vi "Dresden R2R Sputter 03.02.2018 IY24.vi"() -> ()   [LabVIEW 2009] (continued)
                    frame #0 {
                    }
                    frame #1 {
                      # "Hata mesajı"
                      n13036 = local write "Semi"(TRUE ("Semi")) -> ()
                    }
                  }
                  n13037 = local read "Routine_check_transfer"() -> (w19690:bool)
                  n13038 = local read "Semi"() -> (w19692:bool)
                  n13039 = Not(x=w19690) -> (.not. x?=w19691:bool)
                  n13040 = Or(x=w19691, y=w19692) -> (x .or. y?=w19693:bool)
                }
              }
              frame #2 {
                n13041 = Wait (ms)(milliseconds to wait=u32 500) -> ()  [unwired: 1 out]
              }
            }
          }
          frame #2 {
            # "STARTED UP CH3"
            n13042 = disable-structure shown="Disabled" {
              frame #0 {
                n13043 = local read "Semi"() -> (w19700:bool)
                n13044 = case shown="False" w19700 {
                  frame #0 {
                    n13045 = local read "started_up_ch3"() -> (w19701:bool)
                    n13046 = case shown="False" w19701 {
                      frame #0 {
                        n13047 = stacked-sequence {
                          frame #0 {
                            n13048 = local read "Semi"() -> (w19702:bool)
                            n13049 = case shown="False" w19702 {
                              frame #0 {
                                n13050 = local write "Start_up_ch3"(TRUE ("Start_up_ch2")) -> ()
                              }
                              frame #1 {
                              }
                            }
                          }
                          frame #1 {
                            n13051 = local read "Semi"() -> (w19704:bool)
                            n13052 = case shown="False" w19704 {
                              frame #0 {
                                n13053 = Wait (ms)(milliseconds to wait=u32 16000) -> ()  [unwired: 1 out]
                              }
                              frame #1 {
                              }
                            }
                          }
                          frame #2 {
                            n13054 = local read "Semi"() -> (w19706:bool)
                            n13055 = case shown="False" w19706 {
                              frame #0 {
                                n13056 = while {
                                i -> [w19711]
                                stop <- w19708 stop-if-true
                                n13057 = Greater?(x=w19711, y=80) -> (0:w19709:bool)
                                n13058 = local read "started_up_ch3"() -> (w19707:bool)
                                n13059 = case shown="True" w19709 {
                                frame #0 {
                                }
                                frame #1 {
                                n13060 = local write "Semi"(TRUE ("Semi")) -> ()
                                n13061 = local write "Error Message"("Chamber 1 Pressure is not suitable  \nfor transfer process!\nPlease check connections." ("Error Message")) -> ()
                                }
                                }
                                n13062 = case shown="False" w19707 {
                                tunnel: [FALSE TRUE] -> w19708
                                frame #0 {
                                n13063 = Wait Until Next ms Multiple(millisecond multiple=u32 200) -> ()  [unwired: 1 out]
                                }
                                frame #1 {
                                }
                                }
                                }
                              }
                              frame #1 {
                              }
                            }
                          }
                          frame #3 {
                            n13064 = local read "Semi"() -> (w19717:bool)
                            n13065 = case shown="False" w19717 {
                              frame #0 {
                                n13066 = local write "CH1_2_trns_0"(TRUE ("CH1_2_trns_0")) -> ()
                                n13067 = Wait (ms)(milliseconds to wait=u32 1000) -> ()  [unwired: 1 out]
                              }
                              frame #1 {
                              }
                            }
                          }
                        }
                      }
                      frame #1 {
                      }
                    }
                  }
                  frame #1 {
                  }
                }
              }
              frame #1 {
              }
            }
          }
          frame #3 {
            # "STARTED UP CH2"
            n13068 = disable-structure shown="Disabled" {
              frame #0 {
                n13069 = local read "Semi"() -> (w19720:bool)
                n13070 = case shown="False" w19720 {
                  frame #0 {
                    n13071 = local read "started_up_ch2"() -> (w19721:bool)
                    n13072 = case shown="False" w19721 {
                      frame #0 {
                        n13073 = stacked-sequence {
                          frame #0 {
                            n13074 = local read "Semi"() -> (w19722:bool)
                            n13075 = case shown="False" w19722 {
                              frame #0 {
                                n13076 = local write "Start_up_ch2"(TRUE ("Start_up_ch2")) -> ()
                              }
                              frame #1 {
                              }
                            }
                          }
                          frame #1 {
                            n13077 = local read "Semi"() -> (w19724:bool)
                            n13078 = case shown="False" w19724 {
                              frame #0 {
                                n13079 = Wait (ms)(milliseconds to wait=u32 18000) -> ()  [unwired: 1 out]
                              }
                              frame #1 {
                              }
                            }
                          }
                          frame #2 {
                            n13080 = local read "Semi"() -> (w19726:bool)
                            n13081 = case shown="False" w19726 {
                              frame #0 {
                                n13082 = while {
                                i -> [w19731]
                                stop <- w19728 stop-if-true
                                n13083 = Greater?(x=w19731, y=90) -> (0:w19729:bool)
                                n13084 = local read "started_up_ch2"() -> (w19727:bool)
                                n13085 = case shown="True" w19729 {
                                frame #0 {
                                }
                                frame #1 {
                                n13086 = local write "Semi"(TRUE ("Semi")) -> ()
                                n13087 = local write "Error Message"("Chamber 2 Pressure is not suitable  \nfor transfer process!\nPlease check connections." ("Error Message")) -> ()
                                }
                                }
                                n13088 = case shown="False" w19727 {
                                tunnel: [FALSE TRUE] -> w19728
                                frame #0 {
                                n13089 = Wait Until Next ms Multiple(millisecond multiple=u32 200) -> ()  [unwired: 1 out]
                                }
                                frame #1 {
                                }
                                }
                                }
                              }
                              frame #1 {
                              }
                            }
                          }
                          frame #3 {
                            n13090 = local read "Semi"() -> (w19737:bool)
                            n13091 = case shown="False" w19737 {
                              frame #0 {
                                n13092 = local write "CH1_2_trns_1"(TRUE ("CH1_2_trns_0")) -> ()
                                n13093 = Wait (ms)(milliseconds to wait=u32 1000) -> ()  [unwired: 1 out]
                              }
                              frame #1 {
                              }
                            }
                          }
                        }
                      }
                      frame #1 {
                      }
                    }
                  }
                  frame #1 {
                  }
                }
              }
              frame #1 {
              }
            }
          }
          frame #4 {
            # "TRNS GV-BP OPEN"
            n13094 = local read "Semi"() -> (w19740:bool)
            n13095 = case shown="False" w19740 {
              frame #0 {
                n13096 = stacked-sequence {
                  frame #0 {
                    n13097 = local read "Semi"() -> (w19741:bool)
                    n13098 = case shown="False" w19741 {
                      frame #0 {
                        n13099 = while {
                          i -> [w19748]
                          stop <- w19743 stop-if-true
                          n13100 = Greater?(x=w19748, y=50) -> (0:w19746:bool)
                          n13101 = local read "Ch2_trns_gv_bp2_di"() -> (w19742:bool)
                          n13102 = case shown="True" w19746 {
                            frame #0 {
                            }
                            frame #1 {
                              n13103 = local write "Semi"(TRUE ("Semi")) -> ()
                              n13104 = local write "Error Message"("Transfer process was cancelled.\nPlease check CH1-Trns-GV connections." ("Error Message")) -> ()
                            }
                          }
                          n13105 = case shown="False" w19742 {
                            tunnel: [FALSE TRUE] -> w19745
                            frame #0 {
                              n13106 = Wait Until Next ms Multiple(millisecond multiple=u32 200) -> ()  [unwired: 1 out]
                              n13107 = local write "Ch2_trns_gv_bp2_do"(TRUE ("Ch1_pet_cool_up_do")) -> ()
                            }
                            frame #1 {
                            }
                          }
                          n13108 = local read "Semi"() -> (w19744:bool)
                          n13109 = Or(x=w19745, y=w19744) -> (x .or. y?=w19743:bool)
                        }
                      }
                      frame #1 {
                      }
                    }
                  }
                  frame #1 {
                    n13110 = local read "Semi"() -> (w19755:bool)
                    n13111 = case shown="False" w19755 {
                      frame #0 {
                        n13112 = Wait (ms)(milliseconds to wait=u32 500) -> ()  [unwired: 1 out]
                      }
                      frame #1 {
                      }
                    }
                  }
                  frame #2 {
                    n13113 = local read "Semi"() -> (w19757:bool)
                    n13114 = case shown="False" w19757 {
                      frame #0 {
                        n13115 = while {
                          i -> [w19764]
                          stop <- w19759 stop-if-true
                          n13116 = Greater?(x=w19764, y=50) -> (0:w19762:bool)
                          n13117 = local read "Ch3_Trns_gv_bp_di"() -> (w19758:bool)
                          n13118 = case shown="True" w19762 {
                            frame #0 {
                            }
                            frame #1 {
                              n13119 = local write "Semi"(TRUE ("Semi")) -> ()
                              n13120 = local write "Error Message"("Transfer process was cancelled.\nPlease check CH1-Trns-GV connections." ("Error Message")) -> ()
                            }
                          }
                          n13121 = case shown="False" w19758 {
                            tunnel: [FALSE TRUE] -> w19761
                            frame #0 {
                              n13122 = local write "Ch3_Trns_gv_bp_do"(TRUE ("Ch1_pet_cool_up_do")) -> ()
                              n13123 = Wait Until Next ms Multiple(millisecond multiple=u32 200) -> ()  [unwired: 1 out]
                            }
                            frame #1 {
                            }
                          }
                          n13124 = local read "Semi"() -> (w19760:bool)
                          n13125 = Or(x=w19761, y=w19760) -> (x .or. y?=w19759:bool)
                        }
                      }
                      frame #1 {
                      }
                    }
                  }
                  frame #3 {
                    n13126 = local read "Semi"() -> (w19771:bool)
                    n13127 = case shown="False" w19771 {
                      frame #0 {
                        n13128 = Wait (ms)(milliseconds to wait=u32 500) -> ()  [unwired: 1 out]
                      }
                      frame #1 {
                      }
                    }
                  }
                }
              }
              frame #1 {
              }
            }
          }
          frame #5 {
            # "TRNS GV OPEN"
            n13129 = local read "Semi"() -> (w19773:bool)
            n13130 = case shown="False" w19773 {
              frame #0 {
                n13131 = stacked-sequence {
                  frame #0 {
                    n13132 = local read "Semi"() -> (w19774:bool)
                    n13133 = case shown="False" w19774 {
                      frame #0 {
                        n13134 = local write "Ch2_Trns_gv_close_do"(FALSE ("Ch1_pet_cool_up_do")) -> ()
                      }
                      frame #1 {
                      }
                    }
                  }
                  frame #1 {
                    n13135 = local read "Semi"() -> (w19776:bool)
                    n13136 = case shown="False" w19776 {
                      frame #0 {
                        n13137 = while {
                          i -> [w19783]
                          stop <- w19778 stop-if-true
                          n13138 = Greater?(x=w19783, y=500) -> (0:w19781:bool)
                          n13139 = local read "Ch2_Trns_gv_open_di"() -> (w19777:bool)
                          n13140 = case shown="True" w19781 {
                            frame #0 {
                            }
                            frame #1 {
                              n13141 = local write "Semi"(TRUE ("Semi")) -> ()
                              n13142 = local write "Error Message"("Transfer process was cancelled.\nPlease check CH1-Trns-GV connections." ("Error Message")) -> ()
                            }
                          }
                          n13143 = case shown="False" w19777 {
                            tunnel: [FALSE TRUE] -> w19780
                            frame #0 {
                              n13144 = Wait Until Next ms Multiple(millisecond multiple=u32 200) -> ()  [unwired: 1 out]
                              n13145 = local write "Ch2_Trns_gv_open_do"(TRUE ("Ch1_pet_cool_up_do")) -> ()
                            }
                            frame #1 {
                            }
                          }
                          n13146 = local read "Semi"() -> (w19779:bool)
                          n13147 = Or(x=w19780, y=w19779) -> (x .or. y?=w19778:bool)
                        }
                      }
                      frame #1 {
                      }
                    }
                  }
                  frame #2 {
                    n13148 = local read "Semi"() -> (w19790:bool)
                    n13149 = case shown="False" w19790 {
                      frame #0 {
                        n13150 = local write "CH1_2trns_2"(TRUE ("CH1_2trns_5")) -> ()
                        n13151 = Wait (ms)(milliseconds to wait=u32 500) -> ()  [unwired: 1 out]
                      }
                      frame #1 {
                      }
                    }
                  }
                }
              }
              frame #1 {
              }
            }
          }
          frame #6 {
            # "TRNS GV control Trnsgv 2_3"
            n13152 = local read "Semi"() -> (w19793:bool)
            n13153 = case shown="False" w19793 {
              frame #0 {
                n13154 = stacked-sequence {
                  frame #0 {
                    n13155 = local read "Semi"() -> (w19794:bool)
                    n13156 = case shown="False" w19794 {
                      frame #0 {
                        n13157 = while {
                          i -> [w19801]
                          stop <- w19796 stop-if-true
                          n13158 = Greater?(x=w19801, y=50) -> (0:w19799:bool)
                          n13159 = local read "Ch2_TGV_control_di"() -> (w19795:bool)
                          n13160 = case shown="True" w19799 {
                            frame #0 {
                            }
                            frame #1 {
                              n13161 = local write "Semi"(TRUE ("Semi")) -> ()
                              n13162 = local write "Error Message"("Transfer process was cancelled.\nPlease check TRNS-GV connections." ("Error Message")) -> ()
                            }
                          }
                          n13163 = case shown="True" w19795 {
                            tunnel: [TRUE FALSE] -> w19798
                            frame #0 {
                            }
                            frame #1 {
                              n13164 = Wait Until Next ms Multiple(millisecond multiple=u32 200) -> ()  [unwired: 1 out]
                              n13165 = local write "Ch2_TGV_control_do"(FALSE ("Ch1_pet_cool_up_do")) -> ()
                            }
                          }
                          n13166 = local read "Semi"() -> (w19797:bool)
                          n13167 = Or(x=w19798, y=w19797) -> (x .or. y?=w19796:bool)
                        }
                      }
                      frame #1 {
                      }
                    }
                  }
                  frame #1 {
                    n13168 = local read "Semi"() -> (w19808:bool)
                    n13169 = case shown="False" w19808 {
                      frame #0 {
                        n13170 = local write "CH1_2trns_3"(TRUE ("CH1_2trns_5")) -> ()
                        n13171 = Wait (ms)(milliseconds to wait=u32 500) -> ()  [unwired: 1 out]
                      }
                      frame #1 {
                      }
                    }
                  }
                }
              }
              frame #1 {
              }
            }
          }
          frame #7 {
            # "TRNS GV control Trnsgv 2_3"
            n13172 = local read "Semi"() -> (w19811:bool)
            n13173 = case shown="False" w19811 {
              frame #0 {
                n13174 = stacked-sequence {
                  frame #0 {
                    n13175 = local read "Semi"() -> (w19812:bool)
                    n13176 = case shown="False" w19812 {
                      frame #0 {
                        n13177 = while {
                          i -> [w19819]
                          stop <- w19814 stop-if-true
                          n13178 = Greater?(x=w19819, y=50) -> (0:w19817:bool)
                          n13179 = local read "Ch1_Trns_interlock_di"() -> (w19813:bool)
                          n13180 = case shown="True" w19817 {
                            frame #0 {
                            }
                            frame #1 {
                              n13181 = local write "Semi"(TRUE ("Semi")) -> ()
                              n13182 = local write "Error Message"("Transfer process was cancelled.\nPlease check TRNS-GV connections." ("Error Message")) -> ()
                            }
                          }
                          n13183 = case shown="False" w19813 {
                            tunnel: [w19821 TRUE] -> w19816
                            frame #0 {
                              n13184 = local read "Ch1_TGV_control_di"() -> (w19820:bool)
                              n13185 = case shown="False" w19820 {
                                tunnel: [FALSE TRUE] -> w19821
                                frame #0 {
                                n13186 = Wait Until Next ms Multiple(millisecond multiple=u32 200) -> ()  [unwired: 1 out]
                                n13187 = local write "Ch1_TGV_control_do"(TRUE ("Ch1_pet_cool_up_do")) -> ()
                                }
                                frame #1 {
                                }
                              }
                            }
                            frame #1 {
                            }
                          }
                          n13188 = local read "Semi"() -> (w19815:bool)
                          n13189 = Or(x=w19816, y=w19815) -> (x .or. y?=w19814:bool)
                        }
                      }
                      frame #1 {
                      }
                    }
                  }
                  frame #1 {
                    n13190 = local read "Semi"() -> (w19829:bool)
                    n13191 = case shown="False" w19829 {
                      frame #0 {
                        n13192 = local write "CH1_2trns_3"(TRUE ("CH1_2trns_5")) -> ()
                        n13193 = Wait (ms)(milliseconds to wait=u32 500) -> ()  [unwired: 1 out]
                      }
                      frame #1 {
                      }
                    }
                  }
                }
              }
              frame #1 {
              }
            }
          }
          frame #8 {
            # "TRNS GV control Trnsgv 3_4"
            n13194 = local read "Semi"() -> (w19832:bool)
            n13195 = case shown="False" w19832 {
              frame #0 {
                n13196 = stacked-sequence {
                  frame #0 {
                    n13197 = local read "Semi"() -> (w19833:bool)
                    n13198 = case shown="False" w19833 {
                      frame #0 {
                        n13199 = while {
                          i -> [w19840]
                          stop <- w19835 stop-if-true
                          n13200 = Greater?(x=w19840, y=50) -> (0:w19838:bool)
                          n13201 = local read "Ch3_Trns_interlock_di"() -> (w19834:bool)
                          n13202 = case shown="True" w19838 {
                            frame #0 {
                            }
                            frame #1 {
                              n13203 = local write "Semi"(TRUE ("Semi")) -> ()
                              n13204 = local write "Error Message"("Transfer process was cancelled.\nPlease check TRNS-GV connections." ("Error Message")) -> ()
                            }
                          }
                          n13205 = case shown="False" w19834 {
                            tunnel: [w19842 TRUE] -> w19837
                            frame #0 {
                              n13206 = local read "Ch3_TGV_control_di"() -> (w19841:bool)
                              n13207 = case shown="False" w19841 {
                                tunnel: [FALSE TRUE] -> w19842
                                frame #0 {
                                n13208 = Wait Until Next ms Multiple(millisecond multiple=u32 200) -> ()  [unwired: 1 out]
                                n13209 = local write "Ch3_TGV_control_do"(TRUE ("Ch1_pet_cool_up_do")) -> ()
                                }
                                frame #1 {
                                }
                              }
                            }
                            frame #1 {
                            }
                          }
                          n13210 = local read "Semi"() -> (w19836:bool)
                          n13211 = Or(x=w19837, y=w19836) -> (x .or. y?=w19835:bool)
                        }
                      }
                      frame #1 {
                      }
                    }
                  }
                  frame #1 {
                    n13212 = local read "Semi"() -> (w19850:bool)
                    n13213 = case shown="False" w19850 {
                      frame #0 {
                        n13214 = local write "CH1_2trns_4"(TRUE ("CH1_2trns_5")) -> ()
                        n13215 = Wait (ms)(milliseconds to wait=u32 500) -> ()  [unwired: 1 out]
                      }
                      frame #1 {
                      }
                    }
                  }
                }
              }
              frame #1 {
              }
            }
          }
          frame #9 {
            # "Right slow deactive"
            n13216 = local read "Semi"() -> (w19853:bool)
            n13217 = case shown="False" w19853 {
              frame #0 {
                n13218 = stacked-sequence {
                  frame #0 {
                    n13219 = local read "Semi"() -> (w19854:bool)
                    n13220 = case shown="False" w19854 {
                      frame #0 {
                        n13221 = while {
                          i -> [w19857]
                          stop <- w19858 stop-if-true
                          n13222 = Greater?(x=w19857, y=50) -> (0:w19855:bool)
                          n13223 = local read "Cnt_Right_slow_di"() -> (w19861:bool)
                          n13224 = case shown="True" w19855 {
                            frame #0 {
                            }
                            frame #1 {
                              n13225 = local write "Semi"(TRUE ("Semi")) -> ()
                              n13226 = local write "Error Message"("Transfer process was\ncancelled.Please check right slow sensor." ("Error Message")) -> ()
                            }
                          }
                          n13227 = case shown="False" w19861 {
                            tunnel: [FALSE ("Ch1_pet_cool_up_do") TRUE ("Ch1_pet_cool_up_do")] -> w19860
                            frame #0 {
                              n13228 = Wait Until Next ms Multiple(millisecond multiple=u32 200) -> ()  [unwired: 1 out]
                              n13229 = local write "Cnt_Right_slow_do"(TRUE ("Ch1_pet_cool_up_do")) -> ()
                            }
                            frame #1 {
                            }
                          }
                          n13230 = local read "Semi"() -> (w19859:bool)
                          n13231 = Or(x=w19860, y=w19859) -> (x .or. y?=w19858:bool)
                        }
                      }
                      frame #1 {
                      }
                    }
                  }
                  frame #1 {
                    n13232 = local read "Semi"() -> (w19868:bool)
                    n13233 = case shown="False" w19868 {
                      frame #0 {
                        n13234 = local write "CH1_2trns_5"(TRUE ("CH1_2trns_7")) -> ()
                        n13235 = Wait (ms)(milliseconds to wait=u32 500) -> ()  [unwired: 1 out]
                      }
                      frame #1 {
                      }
                    }
                  }
                }
              }
              frame #1 {
              }
            }
          }
          frame #10 {
            # "Right limit deactive"
            n13236 = local read "Semi"() -> (w19871:bool)
            n13237 = case shown="False" w19871 {
              frame #0 {
                n13238 = stacked-sequence {
                  frame #0 {
                    n13239 = local read "Semi"() -> (w19872:bool)
                    n13240 = case shown="False" w19872 {
                      frame #0 {
                        n13241 = while {
                          i -> [w19873]
                          stop <- w19877 stop-if-true
                          n13242 = Greater?(x=w19873, y=50) -> (0:w19875:bool)
                          n13243 = local read "Cnt_Right_limit_di"() -> (w19879:bool)
                          n13244 = case shown="True" w19875 {
                            frame #0 {
                            }
                            frame #1 {
                              n13245 = local write "Semi"(TRUE ("Semi")) -> ()
                              n13246 = local write "Error Message"("Transfer process was\ncancelled.Please check right limit sensor." ("Error Message")) -> ()
                            }
                          }
                          n13247 = case shown="False" w19879 {
                            tunnel: [FALSE ("Ch1_pet_cool_up_do") TRUE ("Ch1_pet_cool_up_do")] -> w19878
                            frame #0 {
                              n13248 = Wait Until Next ms Multiple(millisecond multiple=u32 200) -> ()  [unwired: 1 out]
                              n13249 = local write "Cnt_Right_limit_do"(TRUE ("Ch1_pet_cool_up_do")) -> ()
                            }
                            frame #1 {
                            }
                          }
                          n13250 = local read "Semi"() -> (w19876:bool)
                          n13251 = Or(x=w19878, y=w19876) -> (x .or. y?=w19877:bool)
                        }
                      }
                      frame #1 {
                      }
                    }
                  }
                  frame #1 {
                    n13252 = local read "Semi"() -> (w19886:bool)
                    n13253 = case shown="False" w19886 {
                      frame #0 {
                        n13254 = local write "CH1_2trns_6"(TRUE ("CH1_2trns_7")) -> ()
                        n13255 = Wait (ms)(milliseconds to wait=u32 500) -> ()  [unwired: 1 out]
                      }
                      frame #1 {
                      }
                    }
                  }
                }
              }
              frame #1 {
              }
            }
          }
          frame #11 {
            # "Left slow deactive"
            n13256 = local read "Semi"() -> (w19889:bool)
            n13257 = case shown="False" w19889 {
              frame #0 {
                n13258 = stacked-sequence {
                  frame #0 {
                    n13259 = local read "Semi"() -> (w19890:bool)
                    n13260 = case shown="False" w19890 {
                      frame #0 {
                        n13261 = while {
                          i -> [w19891]
                          stop <- w19895 stop-if-true
                          n13262 = Greater?(x=w19891, y=50) -> (0:w19893:bool)
                          n13263 = local read "Cnt_Left_slow_di"() -> (w19897:bool)
                          n13264 = case shown="True" w19893 {
                            frame #0 {
                            }
                            frame #1 {
                              n13265 = local write "Semi"(TRUE ("Semi")) -> ()
                              n13266 = local write "Error Message"("Transfer process was\ncancelled.Please check left slow sensor." ("Error Message")) -> ()
                            }
                          }
                          n13267 = case shown="False" w19897 {
                            tunnel: [FALSE ("Ch1_pet_cool_up_do") TRUE ("Ch1_pet_cool_up_do")] -> w19896
                            frame #0 {
                              n13268 = Wait Until Next ms Multiple(millisecond multiple=u32 200) -> ()  [unwired: 1 out]
                              n13269 = local write "Cnt_Left_slow_do"(TRUE ("Ch1_pet_cool_up_do")) -> ()
                            }
                            frame #1 {
                            }
                          }
                          n13270 = local read "Semi"() -> (w19894:bool)
                          n13271 = Or(x=w19896, y=w19894) -> (x .or. y?=w19895:bool)
                        }
                      }
                      frame #1 {
                      }
                    }
                  }
                  frame #1 {
                    n13272 = local read "Semi"() -> (w19904:bool)
                    n13273 = case shown="False" w19904 {
                      frame #0 {
                        n13274 = local write "CH1_2trns_7"(TRUE ("CH1_2trns_6b")) -> ()
                        n13275 = Wait (ms)(milliseconds to wait=u32 500) -> ()  [unwired: 1 out]
                      }
                      frame #1 {
                      }
                    }
                  }
                }
              }
              frame #1 {
              }
            }
          }
          frame #12 {
            # "Left limit deactive"
            n13276 = local read "Semi"() -> (w19907:bool)
            n13277 = case shown="False" w19907 {
              frame #0 {
                n13278 = stacked-sequence {
                  frame #0 {
                    n13279 = local read "Semi"() -> (w19908:bool)
                    n13280 = case shown="False" w19908 {
                      frame #0 {
                        n13281 = while {
                          i -> [w19909]
                          stop <- w19913 stop-if-true
                          n13282 = Greater?(x=w19909, y=50) -> (0:w19911:bool)
                          n13283 = local read "Cnt_Left_limit_di"() -> (w19915:bool)
                          n13284 = case shown="True" w19911 {
                            frame #0 {
                            }
                            frame #1 {
                              n13285 = local write "Semi"(TRUE ("Semi")) -> ()
                              n13286 = local write "Error Message"("Transfer process was\ncancelled.Please check left limit sensor." ("Error Message")) -> ()
                            }
                          }
                          n13287 = case shown="False" w19915 {
                            tunnel: [FALSE ("Ch1_pet_cool_up_do") TRUE ("Ch1_pet_cool_up_do")] -> w19914
                            frame #0 {
                              n13288 = Wait Until Next ms Multiple(millisecond multiple=u32 200) -> ()  [unwired: 1 out]
                              n13289 = local write "Cnt_Left_limit_do"(TRUE ("Ch1_pet_cool_up_do")) -> ()
                            }
                            frame #1 {
                            }
                          }
                          n13290 = local read "Semi"() -> (w19912:bool)
                          n13291 = Or(x=w19914, y=w19912) -> (x .or. y?=w19913:bool)
                        }
                      }
                      frame #1 {
                      }
                    }
                  }
                  frame #1 {
                    n13292 = local read "Semi"() -> (w19922:bool)
                    n13293 = case shown="False" w19922 {
                      frame #0 {
                        n13294 = local write "CH1_2trns_8"(TRUE ("CH1_2trns_6c")) -> ()
                        n13295 = Wait (ms)(milliseconds to wait=u32 500) -> ()  [unwired: 1 out]
                      }
                      frame #1 {
                      }
                    }
                  }
                }
              }
              frame #1 {
              }
            }
          }
          frame #13 {
            # "Casette Direction"
            n13296 = local read "Semi"() -> (w19925:bool)
            n13297 = case shown="False" w19925 {
              frame #0 {
                n13298 = stacked-sequence {
                  frame #0 {
                    n13299 = local read "Semi"() -> (w19926:bool)
                    n13300 = case shown="False" w19926 {
                      frame #0 {
                        n13301 = while {
                          i -> [w19932]
                          stop <- w19927 stop-if-true
                          n13302 = Greater?(x=w19932, y=50) -> (0:w19933:bool)
                          n13303 = case shown="True" w19933 {
                            frame #0 {
                            }
                            frame #1 {
                              n13304 = local write "Semi"(TRUE ("Semi")) -> ()
                              n13305 = local write "Error Message"("Transfer process was cancelled.\nPlease check Casette Direction connections." ("Error Message")) -> ()
                            }
                          }
                          n13306 = local read "Casette_servo_left_direction_di"() -> (w19930:bool)
                          n13307 = case shown="True" w19930 {
                            tunnel: [TRUE ("Casette_servo_left_direction_do") FALSE ("Casette_servo_left_direction_do")] -> w19929
                            frame #0 {
                            }
                            frame #1 {
                              n13308 = Wait Until Next ms Multiple(millisecond multiple=u32 200) -> ()  [unwired: 1 out]
                              n13309 = local write "Casette_servo_left_direction_do"(FALSE ("Casette_servo_left_direction_do")) -> ()
                            }
                          }
                          n13310 = local read "Semi"() -> (w19928:bool)
                          n13311 = Or(x=w19929, y=w19928) -> (x .or. y?=w19927:bool)
                        }
                      }
                      frame #1 {
                      }
                    }
                  }
                  frame #1 {
                    n13312 = local read "Semi"() -> (w19940:bool)
                    n13313 = case shown="False" w19940 {
                      frame #0 {
                        n13314 = local write "CH1_2trns_9"(TRUE ("CH1_2trns_7")) -> ()
                        n13315 = Wait (ms)(milliseconds to wait=u32 500) -> ()  [unwired: 1 out]
                      }
                      frame #1 {
                      }
                    }
                  }
                }
              }
              frame #1 {
              }
            }
          }
          frame #14 {
            # "SET CASSETTE SERVO  SPEED 300"
            n13316 = local read "Semi"() -> (w19943:bool)
            n13317 = case shown="False" w19943 {
              frame #0 {
                n13318 = stacked-sequence {
                  frame #0 {
                    n13319 = local read "Semi"() -> (w19944:bool)
                    n13320 = case shown="False" w19944 {
                      frame #0 {
                        n13321 = local write "Cassette_servo_speed_value"(u16 300 ("Cassette_servo_speed_value")) -> ()
                      }
                      frame #1 {
                      }
                    }
                  }
                  frame #1 {
                    n13322 = local read "Semi"() -> (w19946:bool)
                    n13323 = case shown="False" w19946 {
                      frame #0 {
                        n13324 = Wait (ms)(milliseconds to wait=u32 200) -> ()  [unwired: 1 out]
                      }
                      frame #1 {
                      }
                    }
                  }
                  frame #2 {
                    n13325 = local read "Semi"() -> (w19948:bool)
                    n13326 = case shown="False" w19948 {
                      frame #0 {
                        n13327 = local write "Cassette_servo_speed_auto_set"(TRUE ("Cassette_servo_speed_set")) -> ()
                      }
                      frame #1 {
                      }
                    }
                  }
                  frame #3 {
                    n13328 = local read "Semi"() -> (w19950:bool)
                    n13329 = case shown="False" w19950 {
                      frame #0 {
                        n13330 = Wait (ms)(milliseconds to wait=u32 200) -> ()  [unwired: 1 out]
                      }
                      frame #1 {
                      }
                    }
                  }
                  frame #4 {
                    n13331 = local read "Semi"() -> (w19952:bool)
                    n13332 = case shown="False" w19952 {
                      frame #0 {
                        n13333 = local write "CH1_2trns_10"(TRUE ("CH1_2trns_7")) -> ()
                        n13334 = Wait (ms)(milliseconds to wait=u32 500) -> ()  [unwired: 1 out]
                      }
                      frame #1 {
                      }
                    }
                  }
                }
              }
              frame #1 {
              }
            }
          }
          frame #15 {
            # "Casette Servo Start"
            n13335 = local read "Semi"() -> (w19955:bool)
            n13336 = case shown="False" w19955 {
              frame #0 {
                n13337 = stacked-sequence {
                  frame #0 {
                    n13338 = while {
                      i -> [w19961]
                      stop <- w19956 stop-if-true
                      n13339 = Greater?(x=w19961, y=50) -> (0:w19962:bool)
                      n13340 = local read "Casette_servo_start/stop_di"() -> (w19959:bool)
                      n13341 = case shown="True" w19962 {
                        frame #0 {
                        }
                        frame #1 {
                          n13342 = local write "Semi"(TRUE ("Semi")) -> ()
                          n13343 = local write "Error Message"("Transfer process was cancelled.\nPlease check Casette connections." ("Error Message")) -> ()
                        }
                      }
                      n13344 = case shown="False" w19959 {
                        tunnel: [FALSE ("Casette_servo_left_direction_do") TRUE ("Casette_servo_left_direction_do")] -> w19958
                        frame #0 {
                          n13345 = Wait Until Next ms Multiple(millisecond multiple=u32 200) -> ()  [unwired: 1 out]
                          n13346 = local write "Casette_servo_start/stop_do"(TRUE ("Casette_servo_left_direction_do")) -> ()
                        }
                        frame #1 {
                        }
                      }
                      n13347 = local read "Semi"() -> (w19957:bool)
                      n13348 = Or(x=w19958, y=w19957) -> (x .or. y?=w19956:bool)
                    }
                  }
                  frame #1 {
                    n13349 = local read "Semi"() -> (w19969:bool)
                    n13350 = case shown="False" w19969 {
                      frame #0 {
                        n13351 = local write "CH1_2trns_11"(TRUE ("CH1_2trns_9")) -> ()
                        n13352 = Wait (ms)(milliseconds to wait=u32 500) -> ()  [unwired: 1 out]
                      }
                      frame #1 {
                      }
                    }
                  }
                }
              }
              frame #1 {
              }
            }
          }
          frame #16 {
            # "Right sensors activate"
            n13353 = local read "Semi"() -> (w19972:bool)
            n13354 = case shown="False" w19972 {
              frame #0 {
                n13355 = stacked-sequence {
                  frame #0 {
                    n13356 = while {
                      i -> [w19981]
                      stop <- w19977 stop-if-true
                      n13357 = local read "Counter_read_data"() -> (w19974:i16)
                      n13358 = Greater?(x=w19981, y=1500) -> (0:w19980:bool)
                      n13359 = case shown="True" w19980 {
                        frame #0 {
                        }
                        frame #1 {
                          n13360 = local write "Semi"(TRUE ("Semi")) -> ()
                          n13361 = local write "Error Message"("Transfer process was cancelled.\nPlease check Casette & Sensor\nconnections." ("Error Message")) -> ()
                        }
                      }
                      n13362 = Less Or Equal?(x=w19974, y=i16 3000) -> (x <= y?=w19975:bool)
                      n13363 = case shown="False" w19975 {
                        tunnel: [FALSE TRUE] -> w19978
                        frame #0 {
                          n13364 = Wait Until Next ms Multiple(millisecond multiple=u32 200) -> ()  [unwired: 1 out]
                        }
                        frame #1 {
                        }
                      }
                      n13365 = local read "Semi"() -> (w19976:bool)
                      n13366 = Or(x=w19978, y=w19976) -> (x .or. y?=w19977:bool)
                    }
                  }
                  frame #1 {
                    n13367 = while {
                      i -> [w19990]
                      stop <- w19987 stop-if-true